vi "TrackBatchOfImagesWithGPU.vi"(0 "cross size":i32=120, 3 "X Array Input":i32[](array[numeric])=[103], 5 "Cross Thickness":i32=10, 9 "Array Calibration Cluster":T1(array[cluster])=[{"forget"=10, "obj step between slices"=0.1, "Cosine bandpass\nfor Hilbert"=[0.0, 0.010926187, 0.043227285, 0.0954915, 0.16543472, 0.25, 0.34549153, 0.4477358, 0.55226433, 0.6545086, 0.75, 0.83456534, 0.90450853, 0.95677274, 0.9890738, 1.0, 0.98907375, 0.9567727, 0.90450835, 0.8345653, 0.74999994, 0.65450853, 0.55226415, 0.44773582, 0.34549144, 0.25000006, 0.16543463, 0.09549153, 0.043227226, 0.010926217, 0.0, 0.0, 0.0, 0.0, 0.0, 0.0, 0.0, 0.0, 0.0, 0.0, 0.0, 0.0, 0.0, 0.0, 0.0, 0.0, 0.0, 0.0, 0.0, 0.0, 0.0, 0.0, 0.0, 0.0, 0.0, 0.0, 0.0, 0.0, 0.0, 0.0, 0.0, 0.0, 0.0, 0.0, 0.0, 0.0, 0.0, 0.0, 0.0, 0.0, 0.0, 0.0, 0.0, 0.0, 0.0, 0.0, 0.0, 0.0, 0.0, 0.0, 0.0, 0.0, 0.0, 0.0, 0.0, 0.0, 0.0, 0.0, 0.0, 0.0, 0.0, 0.0, 0.0, 0.0, 0.0, 0.0, 0.0, 0.0, 0.0, 0.0, 0.0, 0.0, 0.0, 0.0, 0.0, 0.0, 0.0, 0.0, 0.0, 0.0, 0.0, 0.0, 0.0, 0.0, 0.0, 0.0, 0.0, 0.0, 0.0, 0.0], "r shifted cal ampl"=array100x50[5000 elements], "r-shifted corkscrew cal"=array100x50[5000 elements], "r shifted cal real"=array100x50[5000 elements]}], 11 "Bead Is Good IN":bool[](array[boolean])=[TRUE], 12 "Y Array Input":i32[](array[numeric])=[103], 14 "Array of Images":u8[][][](array[numeric])=array400x200x200[16000000 elements]) -> (4 "Bead Is Good OUT":bool[](array[boolean])=[TRUE], 6 "GPU tracking X":sgl[][](array[numeric])=[[111.98222], [111.94136], [111.866394], [111.74596], [111.56909], [111.35719], [111.10733], [110.8369], [110.52846], [110.19414], [109.85754], [109.52307], [109.189575], [108.86023], [108.56023], [108.28791], [108.04813], [107.8542], [107.682526], [107.573166], [107.50586], [107.48227], [107.49208], [107.55795], [107.6681], [107.815414], [107.98259], [108.18886], [108.41978], [108.64346], [108.922516], [109.1277], [109.36105], [109.568535], [109.77016], [109.91904], [110.03166], [110.12374], [110.169044], [110.12956], [110.04704], [109.95412], [109.797516], [109.56749], [109.322464], [109.01169], [108.659515], [108.29065], [107.87537], [107.493256], [107.0567], [106.60677], [106.228874], [105.82688], [105.4305], [105.074844], [104.747665], [104.45375], [104.23113], [104.02453], [103.86502], [103.788055], [103.69705], [103.69571], [103.74224], [103.806885], [103.898544], [104.04601], [104.203316], [104.34943], [104.53284], [104.69394], [104.882744], [105.02514], [105.1407], [105.2446], [105.308], [105.29668], [105.285324], [105.20174], [105.06968], [104.91222], [104.70184], [104.4219], [104.08912], [103.74295], [103.37244], [102.935295], [102.47367], [102.04646], [101.59453], [101.088005], [100.64656], [100.191444], [99.785065], [99.358475], [99.013535], [98.70897], [98.43903], [98.19031], [98.019485], [97.896706], [97.8068], [97.77524], [97.77259], [97.82318], [97.89526], [98.012085], [98.13559], [98.287544], [98.457115], [98.604546], [98.77586], [98.89298], [99.00852], [99.09027], [99.14229], [99.14186], [99.10187], [99.05939], [98.92539], [98.75957], [98.54906], [98.25993], [97.96763], [97.64464], [97.25098], [96.83731], [96.41509], [95.95466], [95.50255], [95.06288], [94.65112], [94.174164], [93.784836], [93.41963], [93.06384], [92.7852], [92.524124], [92.313324], [92.1648], [92.05137], [91.993835], [91.98616], [92.03104], [92.12036], [92.234886], [92.402695], [92.56262], [92.73822], [92.96175], [93.15148], [93.34769], [93.52924], [93.68433], [93.81467], [93.94579], [93.994644], [94.00526], [93.99018], [93.9174], [93.806], [93.65393], [93.46004], [93.193634], [92.9218], [92.57979], [92.240715], [91.87605], [91.51288], [91.13159], [90.73457], [90.35875], [90.02562], [89.68498], [89.37965], [89.1431], [88.91345], [88.72368], [88.63117], [88.53146], [88.51378], [88.53171], [88.61992], [88.74431], [88.89984], [89.11659], [89.3388], [89.59979], [89.875854], [90.14926], [90.44596], [90.721214], [90.99268], [91.25253], [91.484825], [91.67018], [91.83653], [91.953], [92.00286], [92.01501], [92.00658], [91.94198], [91.81615], [91.66878], [91.47782], [91.25777], [91.007065], [90.73722], [90.42496], [90.15902], [89.88223], [89.58296], [89.34165], [89.115845], [88.91374], [88.73837], [88.61691], [88.55601], [88.514694], [88.549614], [88.609055], [88.735], [88.909256], [89.12585], [89.3861], [89.6934], [90.02026], [90.407646], [90.75013], [91.103905], [91.52437], [91.88941], [92.252625], [92.63097], [92.927284], [93.22749], [93.46109], [93.68758], [93.859406], [93.96161], [94.04938], [94.052155], [94.025665], [93.95174], [93.858475], [93.71265], [93.55252], [93.437325], [93.16719], [92.98062], [92.784805], [92.58888], [92.4143], [92.26122], [92.12206], [92.07706], [92.00729], [92.02084], [92.07329], [92.1948], [92.33276], [92.53406], [92.78928], [93.08535], [93.428276], [93.76366], [94.198555], [94.61577], [95.05928], [95.510666], [95.968], [96.39708], [96.828995], [97.2105], [97.60632], [98.006516], [98.28164], [98.53262], [98.71829], [98.90478], [99.056816], [99.12836], [99.11383], [99.10632], [99.10936], [99.028], [98.98167], [98.793175], [98.63668], [98.403625], [98.34037], [98.103294], [98.05321], [97.86943], [97.83711], [97.80828], [97.805756], [97.83411], [97.88991], [97.98128], [98.23653], [98.458954], [98.6936], [99.02764], [99.355675], [99.76177], [100.184525], [100.6613], [101.08469], [101.614655], [102.0413], [102.48449], [102.93918], [103.357155], [103.74859], [104.07952], [104.41863], [104.6895], [104.97853], [105.03915], [105.20442], [105.25803], [105.31555], [105.29002], [105.222496], [105.15068], [104.97737], [104.8987], [104.727135], [104.59054], [104.33647], [104.18629], [104.02377], [103.91211], [103.79033], [103.720505], [103.70972], [103.721245], [103.74868], [103.84534], [104.01884], [104.2335], [104.46477], [104.760254], [105.07028], [105.43133], [105.788025], [106.19876], [106.62256], [107.04729], [107.48476], [107.88814], [108.2707], [108.65639], [109.01727], [109.296646], [109.52329], [109.75787], [109.92717], [110.03732], [110.118484], [110.16641], [110.084045], [110.00814], [109.87858], [109.71101], [109.549774], [109.372345], [109.0992], [108.879], [108.645935], [108.40287], [108.16335], [107.9711], [107.80571], [107.65991], [107.56433], [107.484276], [107.49236], [107.49719], [107.589516], [107.69519], [107.83682], [108.0541], [108.30353], [108.56494], [108.862], [109.18173], [109.514496], [109.85775], [110.22045], [110.51636], [110.844925], [111.11725], [111.35841], [111.5605], [111.74224], [111.87321], [111.93556]], 8 "Time (ms)":u32=269, 10 "Y Output from GPU":sgl[][](array[numeric])=[[100.02078], [100.19418], [100.34474], [100.52737], [100.72313], [100.9057], [101.12894], [101.30234], [101.50693], [101.70804], [101.864334], [102.057205], [102.24326], [102.3962], [102.5356], [102.67297], [102.785965], [102.87886], [102.94539], [103.01315], [103.092224], [103.13158], [103.17412], [103.21118], [103.25415], [103.27334], [103.32962], [103.38341], [103.42864], [103.55956], [103.63106], [103.73584], [103.86806], [104.04669], [104.26779], [104.46134], [104.721664], [105.00018], [105.2771], [105.54764], [105.85495], [106.16472], [106.51375], [106.80238], [107.095566], [107.38869], [107.65171], [107.927444], [108.13082], [108.32734], [108.46994], [108.58075], [108.654755], [108.69946], [108.69609], [108.655685], [108.59908], [108.50679], [108.37753], [108.22381], [108.08276], [107.92335], [107.744], [107.58732], [107.433044], [107.32801], [107.201035], [107.112526], [107.083755], [107.095375], [107.121086], [107.18843], [107.33879], [107.459404], [107.681564], [107.9283], [108.197716], [108.47565], [108.81435], [109.12399], [109.50108], [109.83769], [110.18041], [110.498985], [110.79605], [111.08653], [111.317], [111.496796], [111.66229], [111.775665], [111.81966], [111.82126], [111.781494], [111.68469], [111.54387], [111.350586], [111.11684], [110.87053], [110.59423], [110.27241], [109.98085], [109.677155], [109.372574], [109.07765], [108.80172], [108.534134], [108.31877], [108.167816], [108.033585], [107.9469], [107.88495], [107.88251], [107.94006], [108.0385], [108.16489], [108.32918], [108.55121], [108.76233], [109.005066], [109.23404], [109.49775], [109.73391], [109.95644], [110.18187], [110.38116], [110.51462], [110.638504], [110.70652], [110.726265], [110.71884], [110.651566], [110.53707], [110.37545], [110.21155], [109.95143], [109.65364], [109.39101], [109.06119], [108.74448], [108.392075], [108.08942], [107.681244], [107.39119], [107.11708], [106.76921], [106.498474], [106.32019], [106.08223], [105.87225], [105.77707], [105.629166], [105.559006], [105.5293], [105.5286], [105.51318], [105.56233], [105.61615], [105.700485], [105.73291], [105.80209], [105.825356], [105.90739], [105.95948], [105.96336], [105.991486], [105.92859], [105.89247], [105.84035], [105.729416], [105.58203], [105.40782], [105.27098], [105.05594], [104.793106], [104.625854], [104.365], [104.0776], [103.862625], [103.50714], [103.28865], [103.126915], [102.789246], [102.564026], [102.417625], [102.16853], [101.98605], [101.773285], [101.69966], [101.60013], [101.390526], [101.24815], [101.119804], [101.017456], [100.91656], [100.79872], [100.65394], [100.61188], [100.44544], [100.35433], [100.16361], [100.00732], [99.83835], [99.664116], [99.477394], [99.32034], [99.10548], [98.93297], [98.73857], [98.49909], [98.3735], [98.15156], [97.961914], [97.84602], [97.646835], [97.49771], [97.397705], [97.23744], [97.24709], [97.07806], [96.91852], [96.90279], [96.852615], [96.83465], [96.80264], [96.82378], [96.7498], [96.72118], [96.64581], [96.613434], [96.49822], [96.386604], [96.27922], [96.12068], [95.948364], [95.77089], [95.54376], [95.34651], [95.07735], [94.77669], [94.45997], [94.212616], [93.85475], [93.54529], [93.24475], [92.91551], [92.63639], [92.404625], [92.164825], [91.941925], [91.733864], [91.59933], [91.49293], [91.39973], [91.37572], [91.32661], [91.39579], [91.4389], [91.58106], [91.67978], [91.82303], [91.957565], [92.15302], [92.298096], [92.49307], [92.62813], [92.77077], [92.84444], [92.92993], [92.969986], [92.97792], [92.92459], [92.84243], [92.70941], [92.550446], [92.33984], [92.09249], [91.81951], [91.53652], [91.199295], [90.84617], [90.5215], [90.179276], [89.83332], [89.50707], [89.22265], [88.92613], [88.7103], [88.50676], [88.357925], [88.25541], [88.17505], [88.17754], [88.23568], [88.33848], [88.47073], [88.67296], [88.89535], [89.151665], [89.43297], [89.71658], [90.04161], [90.3455], [90.64408], [90.95], [91.23329], [91.46195], [91.674194], [91.86136], [91.993546], [92.07825], [92.11565], [92.12019], [92.07689], [91.98989], [91.84635], [91.685936], [91.47246], [91.27072], [91.01648], [90.761116], [90.53021], [90.280685], [90.03856], [89.83711], [89.65035], [89.47775], [89.368965], [89.3099], [89.26545], [89.27579], [89.34183], [89.46566], [89.60816], [89.795456], [90.02495], [90.314285], [90.59569], [90.91796], [91.2439], [91.58194], [91.95044], [92.27831], [92.6248], [92.93144], [93.22364], [93.48745], [93.73809], [93.95398], [94.144226], [94.261215], [94.37112], [94.433914], [94.47505], [94.505806], [94.46933], [94.45236], [94.43618], [94.34592], [94.2929], [94.22064], [94.16539], [94.11157], [94.07608], [94.06795], [94.04411], [94.072105], [94.145294], [94.21954], [94.29191], [94.426346], [94.58866], [94.75017], [94.99471], [95.17778], [95.39114], [95.667496], [95.90499], [96.16127], [96.4372], [96.68062], [96.93535], [97.16527], [97.407036], [97.61966], [97.819756], [98.03491], [98.19011], [98.36585], [98.49895], [98.63775], [98.75882], [98.89068], [99.037155], [99.12136], [99.24571], [99.36879], [99.46666], [99.620544], [99.70962], [99.87132]], 15 "Z from gpu":sgl[][](array[numeric])=[[5.9013395], [5.8662243], [5.8369794], [5.8073306], [5.781902], [5.756898], [5.740077], [5.723185], [5.7105255], [5.6989594], [5.694402], [5.6970024], [5.7068157], [5.7203584], [5.736503], [5.7586417], [5.7824597], [5.8077216], [5.8382034], [5.8743167], [5.8989196], [5.9334483], [5.959512], [5.989463], [6.018897], [6.043241], [6.0595856], [6.0766196], [6.0869293], [6.0939665], [6.097466], [6.0958915], [6.0889144], [6.077285], [6.058838], [6.0442505], [6.021236], [5.990339], [5.956308], [5.9339], [5.900681], [5.873725], [5.835036], [5.803489], [5.7810225], [5.7551174], [5.739356], [5.7219872], [5.707296], [5.7022324], [5.696872], [5.7032447], [5.7046776], [5.7190986], [5.7400002], [5.7589545], [5.7817497], [5.8074126], [5.8386283], [5.8677535], [5.900845], [5.9327784], [5.961533], [5.9919024], [6.0142183], [6.0407624], [6.061966], [6.0767145], [6.08858], [6.0969024], [6.102013], [6.0979877], [6.088992], [6.0797725], [6.057672], [6.0398355], [6.017554], [5.988491], [5.9647117], [5.9320745], [5.902813], [5.871823], [5.8393183], [5.809058], [5.7817354], [5.7571836], [5.7344527], [5.71963], [5.7079782], [5.6999526], [5.702841], [5.702468], [5.7108746], [5.7230005], [5.7369084], [5.7594028], [5.783496], [5.807981], [5.8357506], [5.8703785], [5.901543], [5.9288564], [5.96236], [5.9897647], [6.0132546], [6.0423865], [6.060623], [6.076383], [6.0892735], [6.094893], [6.1005206], [6.097648], [6.0919094], [6.0764236], [6.059755], [6.0424194], [6.016617], [5.994372], [5.9613385], [5.9344935], [5.899382], [5.868843], [5.83497], [5.809433], [5.779991], [5.7585635], [5.7362456], [5.7204356], [5.7091155], [5.7030544], [5.696267], [5.7042036], [5.7096205], [5.718922], [5.736815], [5.7599273], [5.7818556], [5.810293], [5.8361597], [5.870059], [5.902242], [5.9314504], [5.9593725], [5.991966], [6.0168753], [6.0414042], [6.061048], [6.073913], [6.0894213], [6.095019], [6.097249], [6.0945992], [6.0885224], [6.0721545], [6.056149], [6.042106], [6.016165], [5.9876294], [5.9593883], [5.930475], [5.904896], [5.8685675], [5.8340135], [5.8065805], [5.7813168], [5.7561164], [5.738132], [5.7195306], [5.7083416], [5.70246], [5.6976676], [5.702623], [5.708123], [5.7197037], [5.739213], [5.7573576], [5.781855], [5.8090305], [5.8370104], [5.867156], [5.9010158], [5.932455], [5.9607625], [5.9916863], [6.0177684], [6.0401745], [6.063718], [6.0762672], [6.0888934], [6.097215], [6.0972686], [6.093936], [6.086149], [6.077937], [6.0611663], [6.0406103], [6.015375], [5.9909725], [5.9619365], [5.934942], [5.9013653], [5.869026], [5.837444], [5.805542], [5.784716], [5.7568216], [5.7363024], [5.7164397], [5.7093544], [5.6985364], [5.699764], [5.701771], [5.706639], [5.718078], [5.7357955], [5.7543178], [5.7827563], [5.8074775], [5.8355055], [5.86835], [5.9006786], [5.9292226], [5.963678], [5.989457], [6.0153446], [6.0399394], [6.0636415], [6.07615], [6.086099], [6.097633], [6.096236], [6.0944996], [6.088367], [6.0749], [6.058119], [6.0393014], [6.0197387], [5.9900002], [5.9599733], [5.935629], [5.8982615], [5.868896], [5.834993], [5.8122506], [5.7813687], [5.7580147], [5.7390175], [5.7207856], [5.7113457], [5.7054935], [5.699217], [5.702978], [5.7097774], [5.7191367], [5.7356114], [5.758533], [5.7820625], [5.8059363], [5.8369427], [5.868797], [5.904074], [5.9323206], [5.960735], [5.9914145], [6.0138526], [6.039195], [6.0627437], [6.0757804], [6.091232], [6.0981016], [6.099422], [6.097309], [6.0859914], [6.076905], [6.06256], [6.040302], [6.017345], [5.9898677], [5.9622684], [5.9295964], [5.900269], [5.8707914], [5.8384027], [5.8108635], [5.7829523], [5.7584834], [5.7401443], [5.7223597], [5.7124686], [5.700731], [5.6985984], [5.698714], [5.7111726], [5.7229285], [5.7378745], [5.758489], [5.780324], [5.8103447], [5.8346143], [5.869102], [5.90438], [5.935668], [5.964738], [5.9943385], [6.0180106], [6.0416408], [6.0632753], [6.079457], [6.0892134], [6.0923624], [6.0996103], [6.0957494], [6.0904846], [6.079738], [6.061401], [6.038819], [6.0165615], [5.98843], [5.962503], [5.932745], [5.8998694], [5.868017], [5.8372245], [5.810103], [5.782851], [5.762548], [5.7403746], [5.7197866], [5.7084665], [5.70023], [5.702631], [5.7014546], [5.709451], [5.7179413], [5.737244], [5.759624], [5.778131], [5.807871], [5.836637], [5.864694], [5.8965926], [5.9291134], [5.9626703], [5.989478], [6.019633], [6.0390897], [6.0614467], [6.077993], [6.088981], [6.096026], [6.0982285], [6.0970697], [6.091824], [6.0783095], [6.057942], [6.0422206], [6.0179944], [5.9910483], [5.963313], [5.92998], [5.8963003], [5.867696], [5.8370895], [5.811132], [5.7815614], [5.7584863], [5.737567], [5.7221985], [5.710052], [5.703836], [5.7003403], [5.7028093], [5.7037], [5.7202544], [5.7370067], [5.758294], [5.781157], [5.8136516], [5.838899], [5.869066], [5.9013677], [5.9326444], [5.960175], [5.989266], [6.015803], [6.0397453], [6.061123], [6.072538], [6.089087], [6.097654], [6.096904], [6.095035], [6.0880733], [6.080462], [6.0610914], [6.0399776], [6.012885], [5.9893565], [5.961964], [5.9318023]])   [LabVIEW 2014]
uses:
  x64/Release/GPU Tracking.dll
panel:
  in  "Threads":i32=512
  out "x-y":sgl[][](array[numeric])=[[-147.80074], [-147.8427], [-147.91708], [-148.03627], [-148.21384], [-148.42784], [-148.677], [-148.94637], [-149.25612], [-149.58842], [-149.92584], [-150.2609], [-150.59155], [-150.9241], [-151.22298], [-151.496], [-151.73483], [-151.92693], [-152.09717], [-152.20616], [-152.27188], [-152.29465], [-152.28285], [-152.21771], [-152.10834], [-151.95778], [-151.78966], [-151.58406], [-151.35269], [-151.12827], [-150.8494], [-150.64278], [-150.41049], [-150.20428], [-150.00145], [-149.8529], [-149.74074], [-149.64926], [-149.60373], [-149.64458], [-149.72606], [-149.81932], [-149.97754], [-150.20839], [-150.45387], [-150.76553], [-151.11795], [-151.49011], [-151.90506], [-152.28821], [-152.72684], [-153.17953], [-153.55673], [-153.95898], [-154.35814], [-154.71251], [-155.0421], [-155.3368], [-155.5575], [-155.76465], [-155.92337], [-155.99994], [-156.08838], [-156.0906], [-156.04175], [-155.9754], [-155.8831], [-155.73093], [-155.57349], [-155.42502], [-155.2442], [-155.0817], [-154.8902], [-154.74838], [-154.63335], [-154.52982], [-154.467], [-154.4788], [-154.49193], [-154.5761], [-154.70773], [-154.86617], [-155.0802], [-155.357], [-155.6903], [-156.03696], [-156.40701], [-156.84494], [-157.30414], [-157.73119], [-158.18431], [-158.68939], [-159.13322], [-159.58658], [-159.9902], [-160.41725], [-160.76216], [-161.0709], [-161.33884], [-161.58609]]
  in  "GPU tracking X 2":sgl[][](array[numeric])=[[259.78296, 138.92928, 91.836395, 335.83517, 201.1554, 213.00905, 302.24893, 273.92642], [259.78406, 138.92902, 91.83962, 335.8386, 201.13281, 213.01207, 302.26337, 273.91797], [259.78348, 138.92856, 91.835495, 335.83682, 201.11922, 213.0119, 302.2586, 273.89597], [259.78223, 138.92694, 91.83724, 335.83676, 201.14786, 213.01036, 302.24814, 273.90912], [259.78293, 138.92815, 91.837296, 335.837, 201.16449, 213.01495, 302.24777, 273.9324], [259.78503, 138.92726, 91.84008, 335.8381, 201.19228, 213.01015, 302.2342, 273.93335], [259.78433, 138.9266, 91.84003, 335.83746, 201.18456, 213.01395, 302.22452, 273.89154], [259.78326, 138.92523, 91.837265, 335.8371, 201.19539, 213.01257, 302.21933, 273.89957], [259.78458, 138.92633, 91.840614, 335.8373, 201.2018, 213.01262, 302.24484, 273.92422], [259.78256, 138.9272, 91.839005, 335.8369, 201.17986, 213.00626, 302.25146, 273.92813], [259.7834, 138.93158, 91.8416, 335.83667, 201.1795, 213.01561, 302.2484, 273.92703], [259.78397, 138.92517, 91.83989, 335.83615, 201.15607, 213.01692, 302.2439, 273.93802], [259.78113, 138.92577, 91.83997, 335.8387, 201.11432, 213.01646, 302.2512, 273.9515], [259.78433, 138.92638, 91.837036, 335.83963, 201.11139, 213.01488, 302.26288, 273.95242], [259.7832, 138.92786, 91.841995, 335.8345, 201.13403, 213.01347, 302.25555, 273.93423], [259.7839, 138.92688, 91.83873, 335.83545, 201.14554, 213.0138, 302.24084, 273.9345], [259.78296, 138.92613, 91.84163, 335.8359, 201.17102, 213.01416, 302.21094, 273.91467], [259.78113, 138.92444, 91.83614, 335.83298, 201.1742, 213.0159, 302.18216, 273.9174], [259.7797, 138.92337, 91.83948, 335.8349, 201.1685, 213.01408, 302.16016, 273.9238], [259.77933, 138.92458, 91.84062, 335.8334, 201.17175, 213.01363, 302.1845, 273.9279], [259.77774, 138.92497, 91.837616, 335.83218, 201.1886, 213.00577, 302.2157, 273.9431], [259.77692, 138.9215, 91.83508, 335.83102, 201.16605, 213.00217, 302.22015, 273.9289], [259.77493, 138.92354, 91.83542, 335.83115, 201.19281, 213.00688, 302.21426, 273.9251], [259.77567, 138.92276, 91.8324, 335.8316, 201.17432, 213.00752, 302.21808, 273.94254], [259.77643, 138.91899, 91.83426, 335.82904, 201.16257, 213.00655, 302.21964, 273.9469], [259.7732, 138.92314, 91.83146, 335.82794, 201.1649, 213.00946, 302.21298, 273.93607], [259.77225, 138.9197, 91.83242, 335.83, 201.1627, 213.00514, 302.19864, 273.94934], [259.77292, 138.91881, 91.83327, 335.8276, 201.16055, 213.00668, 302.19693, 273.9381], [259.77246, 138.91628, 91.82982, 335.82727, 201.1822, 213.00453, 302.1962, 273.94086], [259.77173, 138.92014, 91.82837, 335.8254, 201.19144, 213.00761, 302.19293, 273.95352], [259.7719, 138.91899, 91.82772, 335.8258, 201.19403, 213.00697, 302.18298, 273.9429], [259.77048, 138.91716, 91.82741, 335.82596, 201.1927, 213.00351, 302.1855, 273.9445], [259.77155, 138.91711, 91.82643, 335.82443, 201.1682, 212.99905, 302.16745, 273.95718], [259.77283, 138.91933, 91.830414, 335.82516, 201.14401, 212.99852, 302.13858, 273.95834], [259.7716, 138.91954, 91.82568, 335.82513, 201.16158, 212.99738, 302.15073, 273.94528], [259.77194, 138.9188, 91.82836, 335.82797, 201.14954, 212.99814, 302.1499, 273.93195], [259.7724, 138.92146, 91.82826, 335.82553, 201.13937, 213.00342, 302.1247, 273.92065], [259.773, 138.9197, 91.82702, 335.82706, 201.1388, 212.99762, 302.1199, 273.92648], [259.77277, 138.91714, 91.827515, 335.83038, 201.14929, 213.0076, 302.15137, 273.94107], [259.77414, 138.92091, 91.82726, 335.8278, 201.1308, 213.00975, 302.15732, 273.9348], [259.7731, 138.91905, 91.82978, 335.82626, 201.09412, 213.007, 302.16382, 273.9326], [259.77344, 138.91939, 91.82576, 335.82904, 201.11891, 213.00584, 302.13934, 273.94223], [259.77505, 138.91978, 91.82989, 335.827, 201.11473, 213.00562, 302.1494, 273.963], [259.77588, 138.92036, 91.83061, 335.8286, 201.10078, 213.00735, 302.14325, 273.98508], [259.77634, 138.9249, 91.828896, 335.82758, 201.11792, 213.0068, 302.13806, 273.99734], [259.77722, 138.92294, 91.82943, 335.83112, 201.13275, 213.01349, 302.15848, 273.98935], [259.77747, 138.92418, 91.82882, 335.83472, 201.11412, 213.01527, 302.16742, 273.97647], [259.78076, 138.92448, 91.831154, 335.83194, 201.13527, 213.01387, 302.18488, 273.97073], [259.78043, 138.92657, 91.83212, 335.8351, 201.14581, 213.00781, 302.19095, 273.96518], [259.78146, 138.9253, 91.834915, 335.8377, 201.14542, 213.01324, 302.1907, 273.95], [259.78354, 138.9285, 91.8369, 335.8354, 201.15869, 213.01613, 302.20938, 273.96646], [259.78632, 138.92987, 91.84028, 335.83905, 201.1381, 213.0198, 302.22687, 273.97003], [259.7856, 138.93228, 91.838776, 335.8399, 201.13925, 213.0162, 302.2399, 273.97638], [259.78586, 138.9314, 91.840805, 335.84238, 201.15419, 213.01791, 302.24484, 273.9528], [259.78864, 138.93356, 91.841034, 335.84122, 201.16248, 213.02052, 302.23514, 273.94858], [259.78735, 138.93341, 91.84434, 335.84015, 201.16263, 213.02026, 302.24036, 273.96545], [259.78976, 138.93323, 91.84192, 335.84235, 201.17938, 213.02303, 302.22028, 273.97165], [259.79056, 138.93437, 91.84597, 335.84183, 201.1833, 213.02377, 302.2308, 273.97], [259.78864, 138.93254, 91.84289, 335.8435, 201.19391, 213.0297, 302.22272, 273.94736], [259.78918, 138.93188, 91.84373, 335.8437, 201.20842, 213.01836, 302.24112, 273.94922], [259.7884, 138.93173, 91.844734, 335.84103, 201.19257, 213.0206, 302.2601, 273.93372], [259.788, 138.93106, 91.8435, 335.8411, 201.17868, 213.02261, 302.25287, 273.9155], [259.78543, 138.93216, 91.843895, 335.83905, 201.17789, 213.02336, 302.24948, 273.9086], [259.78632, 138.92705, 91.84534, 335.838, 201.18643, 213.02219, 302.2281, 273.91168], [259.784, 138.92773, 91.83884, 335.83636, 201.19217, 213.02414, 302.22922, 273.92624], [259.7823, 138.92741, 91.83956, 335.83615, 201.20207, 213.0223, 302.22556, 273.9427], [259.78165, 138.92719, 91.8384, 335.83508, 201.2111, 213.01614, 302.2155, 273.95493], [259.77695, 138.92474, 91.842415, 335.83362, 201.19795, 213.01256, 302.17645, 273.93018], [259.7768, 138.92401, 91.83627, 335.8302, 201.16461, 213.0165, 302.16034, 273.92923], [259.77444, 138.92001, 91.83168, 335.83096, 201.17653, 213.01707, 302.15988, 273.93524], [259.77704, 138.92197, 91.8325, 335.827, 201.13681, 213.01065, 302.15222, 273.95145], [259.77563, 138.91805, 91.83065, 335.82883, 201.15068, 213.00433, 302.1497, 273.927], [259.77295, 138.92004, 91.831894, 335.8256, 201.16032, 213.00813, 302.1732, 273.91797], [259.77353, 138.92172, 91.82958, 335.82867, 201.13838, 213.00766, 302.18256, 273.92615], [259.77405, 138.91931, 91.8307, 335.82922, 201.13274, 213.00687, 302.16312, 273.9163], [259.7744, 138.91948, 91.833, 335.82956, 201.13785, 213.01219, 302.18753, 273.93466], [259.775, 138.91931, 91.83379, 335.8293, 201.14635, 213.01372, 302.20728, 273.93848], [259.77548, 138.91943, 91.83053, 335.82788, 201.14188, 213.012, 302.21802, 273.95026], [259.77725, 138.92284, 91.83391, 335.83002, 201.16402, 213.00946, 302.24496, 273.9553], [259.77783, 138.92264, 91.83368, 335.83078, 201.17691, 213.01376, 302.24313, 273.9472], [259.7774, 138.92279, 91.83195, 335.83, 201.16756, 213.01485, 302.21008, 273.94012], [259.77838, 138.92413, 91.83514, 335.83014, 201.16846, 213.01479, 302.2229, 273.95877], [259.78204, 138.92647, 91.835365, 335.82898, 201.17715, 213.0142, 302.2368, 273.96652], [259.7789, 138.9249, 91.83501, 335.83365, 201.1637, 213.01189, 302.26868, 273.94678], [259.77942, 138.92557, 91.83554, 335.8336, 201.15988, 213.01195, 302.27084, 273.9384], [259.7799, 138.92491, 91.834274, 335.83334, 201.146, 213.01509, 302.29138, 273.95645], [259.77945, 138.92543, 91.83588, 335.83258, 201.15442, 213.0164, 302.30334, 273.93823], [259.78024, 138.92465, 91.83458, 335.8321, 201.14507, 213.01439, 302.2681, 273.92822], [259.7778, 138.92401, 91.83493, 335.83102, 201.13419, 213.01553, 302.23465, 273.93494], [259.77765, 138.9255, 91.83325, 335.83218, 201.14671, 213.01065, 302.2181, 273.93546], [259.77884, 138.92332, 91.83191, 335.83276, 201.13347, 213.00877, 302.22144, 273.9462], [259.7774, 138.92645, 91.83311, 335.8316, 201.1324, 213.00627, 302.19995, 273.9647], [259.7798, 138.92622, 91.82913, 335.8324, 201.10638, 213.00702, 302.191, 273.95798], [259.778, 138.92168, 91.831406, 335.82996, 201.13586, 213.00806, 302.18613, 273.937], [259.77527, 138.92302, 91.83217, 335.83078, 201.1399, 213.01268, 302.21384, 273.96735], [259.77573, 138.92137, 91.8293, 335.82834, 201.15562, 213.00932, 302.2131, 273.95575], [259.7757, 138.92401, 91.83184, 335.83017, 201.15578, 213.01155, 302.21445, 273.95032], [259.77988, 138.92233, 91.83262, 335.83005, 201.18744, 213.01204, 302.23563, 273.93484], [259.77786, 138.92323, 91.83183, 335.83008, 201.19339, 213.01456, 302.23776, 273.92288], [259.7764, 138.9251, 91.82976, 335.8316, 201.18959, 213.01643, 302.21664, 273.91418]]
  in  "error in (no error)":errorcluster
  in  "DIM3":i32=1
  in  "DIM4":i32=1
  in  "DIM1":i32=1
  in  "DIM2":i32=1
  out "error out":errorcluster
  out "Error Message":string="No_Errors"
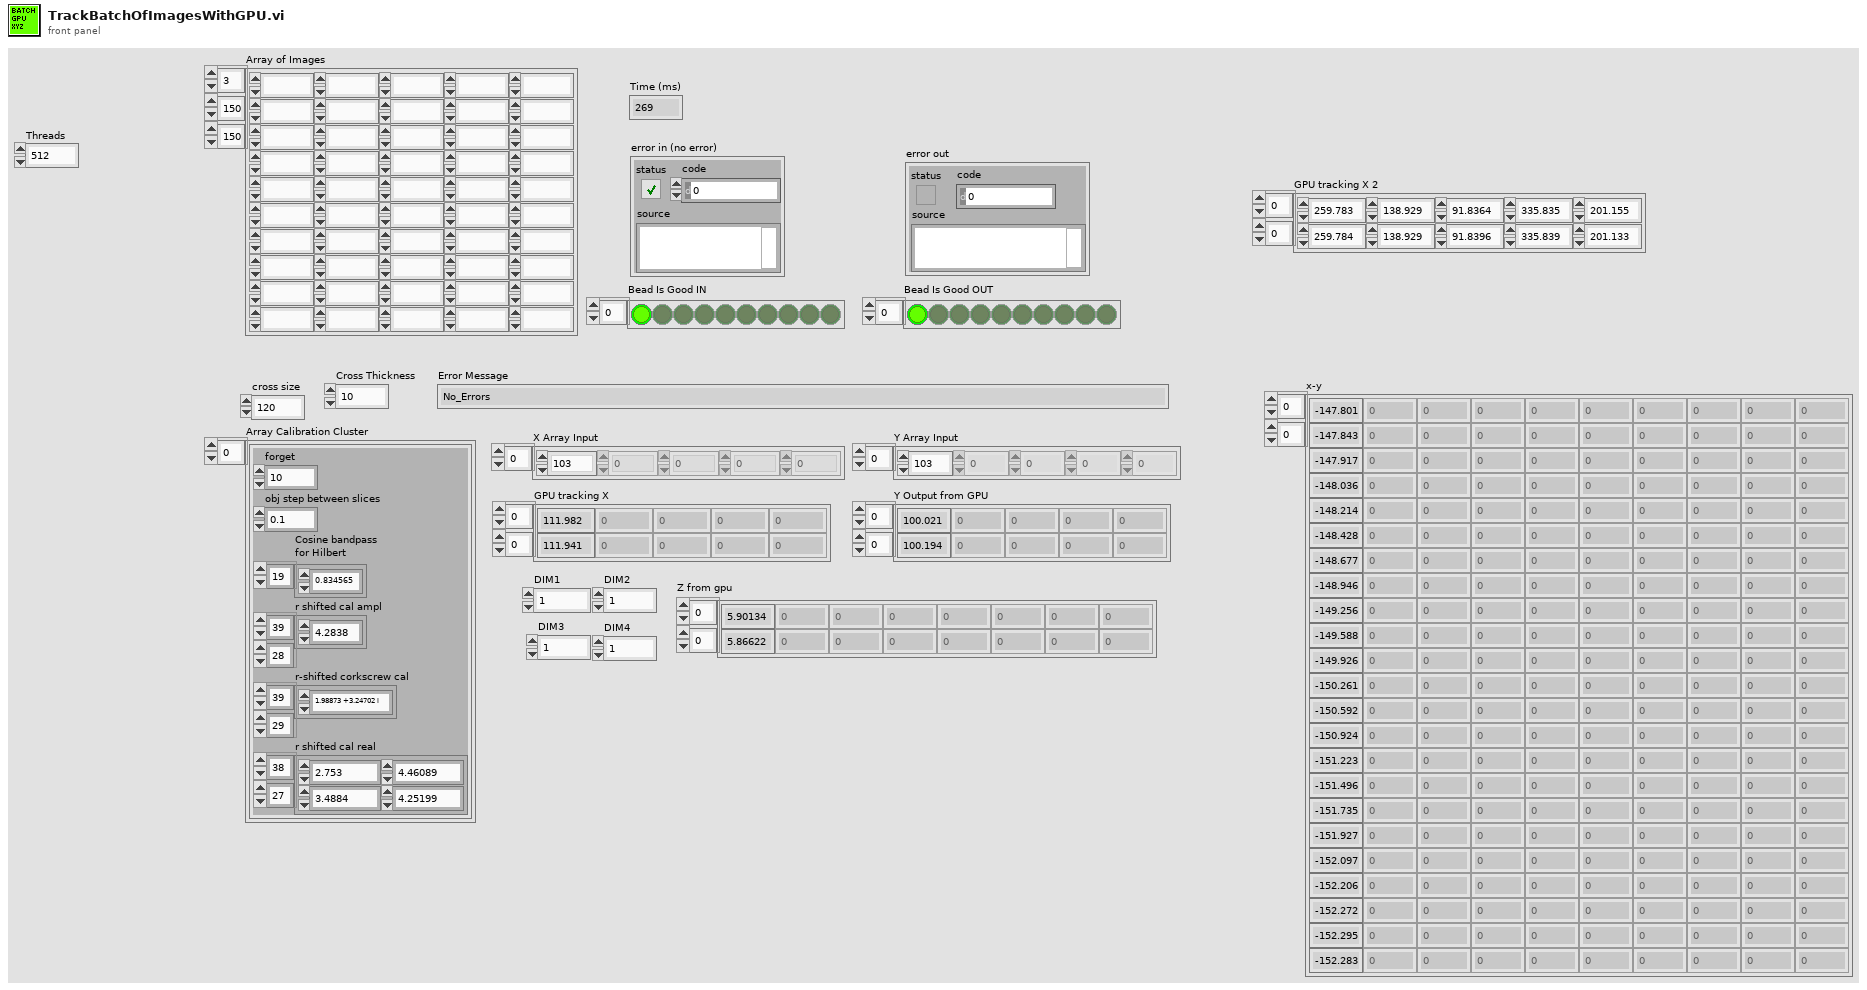
[diagram p1: front panel]
types:
  T1 = cluster{"forget":i32, "obj step between slices":sgl, "Cosine bandpass\nfor Hilbert":sgl[], "r shifted cal ampl":sgl[][], "r-shifted corkscrew cal":csg[][], "r shifted cal real":sgl[][]}[]
  T2 = cluster{"forget":i32, "obj step between slices":sgl, "Cosine bandpass\nfor Hilbert":sgl[], "r shifted cal ampl":sgl[][], "r-shifted corkscrew cal":csg[][], "r shifted cal real":sgl[][]}
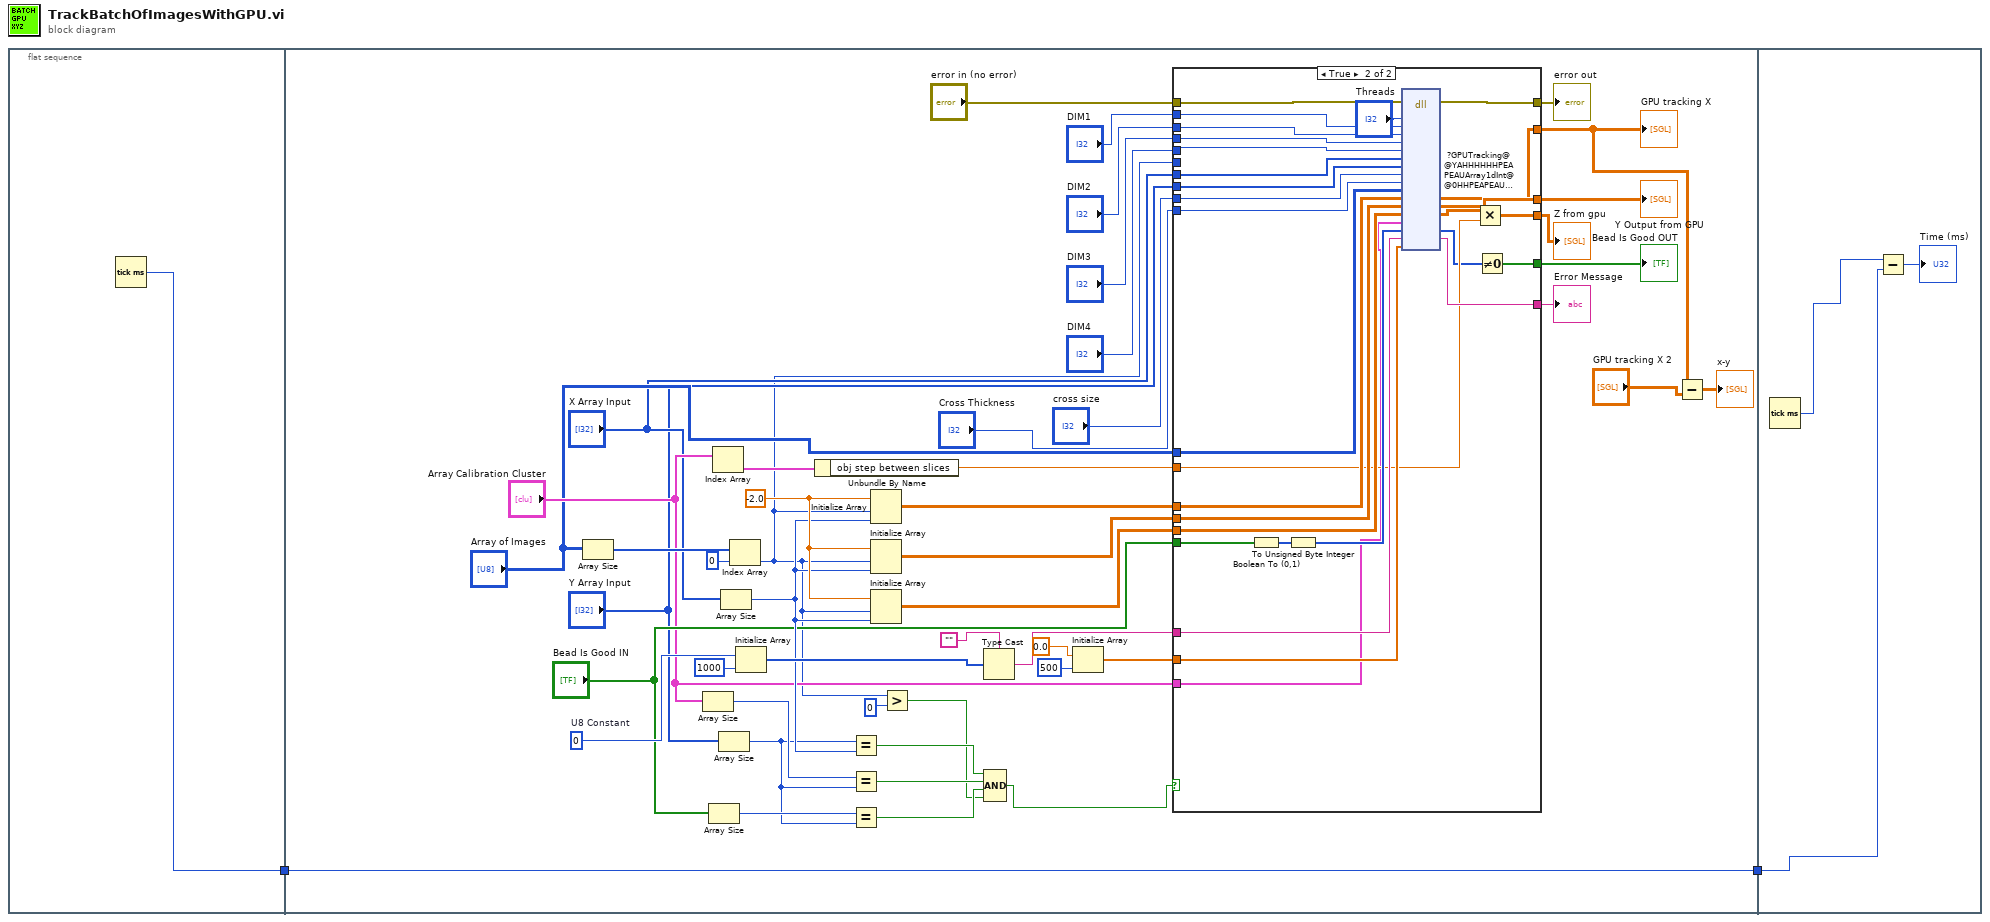
[diagram p0: block diagram]
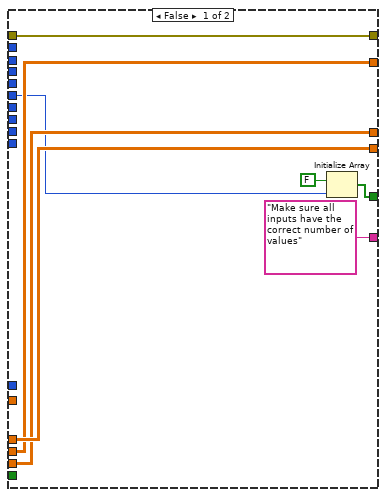
[diagram p2: hidden frame]
diagram:
  n1 = flat-sequence {
    tunnel: [w3] -> w1
    tunnel: [w51] -> w2
    tunnel: w1 -> [w51]
    tunnel: w2 -> [w91]
    frame #0 {
      n2 = Tick Count (ms)() -> (millisecond timer value=w3:u32)
    }
    frame #1 {
      w44 = u8 0  # U8 Constant
      w45 = sgl -2.0 ("element")
      n3 = Array Size(array="Array of Images") -> (size(s)=w50:i32[])
      n4 = Array Size(array="Array Calibration Cluster") -> (size(s)=w34:i32)
      n5 = Array Size(array="Bead Is Good IN") -> (size(s)=w31:i32)
      n6 = Index Array(array="Array Calibration Cluster") -> (element=w25:T2)  [unwired: 1 in]
      n7 = Array Size(array="Y Array Input") -> (size(s)=w30:i32)
      n8 = Array Size(array="X Array Input") -> (size(s)=w35:i32)
      n9 = Index Array(array=w50, index=0) -> (element=w12:i32)
      n10 = Initialize Array(w44, 1000 ("dimension size")) -> (w43:u8[])
      n11 = Unbundle By Name(w25) -> ("obj step between slices"=w24:sgl)
      n12 = Equal?(x=w30, y=w35) -> (x = y?=w36:bool)
      n13 = Equal?(x=w34, y=w30) -> (x = y?=w33:bool)
      n14 = Equal?(x=w31, y=w30) -> (x = y?=w29:bool)
      n15 = Initialize Array(w45, w12, w35) -> (w48:sgl[][])
      n16 = Initialize Array(w45, w12, w35) -> (w49:sgl[][])
      n17 = Initialize Array(w45, w12, w35) -> (w46:sgl[][])
      n18 = Greater?(x=w12, y=0) -> (0:w18:bool)
      n19 = Type Cast(type="", x=w43) -> (*(type *) &x=w40:string)
      n20 = Compound Arithmetic op=AND(w36, w33, w29, w18) -> (w7:bool)
      n21 = Initialize Array(sgl 0.0 ("element"), 500 ("dimension size")) -> (w28:sgl[])
      n22 = case shown="True" w7 {
        tunnel: "cross size" -> [_ w87]
        tunnel: "Y Array Input" -> [_ w76]
        tunnel: "X Array Input" -> [_ w77]
        tunnel: w49 -> [w57 w84]
        tunnel: w48 -> [w58 w85]
        tunnel: "Cross Thickness" -> [_ w86]
        tunnel: w46 -> [w56 w83]
        tunnel: w40 -> [_ w80]
        tunnel: "Array Calibration Cluster" -> [_ w61]
        tunnel: ["Make sure all inputs have the correct number of values" w79] -> w38
        tunnel: [w58 w69] -> w21
        tunnel: [w56 w70] -> w20
        tunnel: [w57 w68] -> w6
        tunnel: "Array of Images" -> [_ w74]
        tunnel: "Bead Is Good IN" -> [_ w75]
        tunnel: [w52 w66] -> w37
        tunnel: w28 -> [_ w81]
        tunnel: w24 -> [_ w78]
        tunnel: "error in (no error)" -> [w55 w73]
        tunnel: [w55 w72] -> w13
        tunnel: w12 -> [w53 _]
        tunnel: "DIM1" -> [_ w65]
        tunnel: "DIM2" -> [_ w64]
        tunnel: "DIM3" -> [_ w63]
        tunnel: "DIM4" -> [_ w62]
        frame False {
          n23 = Initialize Array(FALSE, w53) -> (w52:bool[])
        }
        frame True {
          n24 = Boolean To (0,1)(Boolean=w75) -> (0, 1=w88:i16[])
          n25 = To Unsigned Byte Integer(number=w88) -> (unsigned 8bit integer=w82:u8[])
          n26 = dll-call lib="D:/LV-SVN/Projects/Bob/GPU Tracking Demo/GPU Tracking/x64/Release/GPU Tracking.dll" fn="?GPUTracking@@YAHHHHHHPEAPEAUArray1dInt@@0HHPEAPEAUImage@@PEAPEAUArray2d@@22PEAPEAUArrayCluster@@PEAPEAUBoolArray@@PEADPEAPEAUArray1d@@@Z"(error in=w73, "Threads"="Threads", "DIM1"=w65, "DIM2"=w64, "DIM3"=w63, "DIM4"=w62, "X Array"=w77, "Y Array"=w76, "Cross Size"=w87, "Cross Thickness"=w86, "Array of Images"=w74, "X Output"=w85, "Y Output"=w84, "Z Output"=w83, "Array Cal Cluster"=w61, "Bead Is Good Array"=w82, "Error Message"=w80, "Test Array"=w81) -> (error out=w72:errorcluster, "X Output"=w68:sgl[][], "Y Output"=w70:sgl[][], "Z Output"=w71:sgl[][], "Bead Is Good Array"=w67:u8[], "Error Message"=w79:string)  [unwired: 15 in, 1 out]
          n27 = Multiply(x=w71, y=w78) -> (x*y=w69:sgl[][])
          n28 = Not Equal To 0?(x=w67) -> (x != 0?=w66:bool[])
        }
      }
      "Error Message" <- w38
      "Z from gpu" <- w21
      "Y Output from GPU" <- w20
      "GPU tracking X" <- w6
      "Bead Is Good OUT" <- w37
      "error out" <- w13
      n29 = Subtract(x=w6, y="GPU tracking X 2") -> (x-y=→"x-y":sgl[][])
    }
    frame #2 {
      n30 = Tick Count (ms)() -> (millisecond timer value=w90:u32)
      n31 = Subtract(x=w90, y=w91) -> (x-y=→"Time (ms)":u32)
    }
  }
